vi "FlexMag - 24-03-2023.vi"() -> ()   [LabVIEW 2018] (continued)
                              n10246 = local read "ABORT"() -> (w15652:bool)
                              n10247 = Not(x=w15653) -> (.not. x?=w15651:bool)
                              n10248 = Compound Arithmetic op=OR(w15646, w15652, w15651) -> (w15650:bool)
                            }
                          }
                          frame #2 {
                            n10249 = flat-sequence {
                              frame #0 {
                                n10250 = local write "Cassette_Servo_Speed AO"(0.0 ("Cassette_Servo_Speed AO")) -> ()
                                n10251 = Wait (ms)(milliseconds to wait=u32 100) -> ()  [unwired: 1 out]
                              }
                              frame #1 {
                                n10252 = local write "Cassette_Servo_Speed Set"(TRUE ("Cassette_Servo_Speed Set")) -> ()
                              }
                            }
                          }
                        }
                      }
                      frame True {
                      }
                    }
                  }
                }
              }
              frame #37 {
                n10253 = local read "ch3-4 transfer"() -> (w15663:bool)
                n10254 = case shown="True" w15663 {
                  frame False {
                  }
                  frame True {
                    n10255 = local read "ABORT"() -> (w15664:bool)
                    n10256 = case shown="False" w15664 {
                      frame False {
                        n10257 = local write "trns 3-4 led 17"(TRUE ("trns 1-2 led 1")) -> ()
                        n10258 = Wait (ms)(milliseconds to wait=u32 100) -> ()  [unwired: 1 out]
                      }
                      frame True {
                      }
                    }
                  }
                }
              }
              frame #38 {
                n10259 = local read "ch3-4 transfer"() -> (w15667:bool)
                n10260 = case shown="True" w15667 {
                  frame False {
                  }
                  frame True {
                    n10261 = local read "ABORT"() -> (w15668:bool)
                    n10262 = case shown="False" w15668 {
                      frame False {
                        n10263 = local read "target chamber"() -> (w15669:dbl)
                        n10264 = Equal?(x=w15669, y=4.0) -> (x = y?=w15670:bool)
                        n10265 = case shown="True" w15670 {
                          frame False {
                          }
                          frame True {
                            n10266 = while {
                              i -> [w15676]
                              stop <- w15677 stop-if-true
                              n10267 = Greater Or Equal?(x=w15676, y=100) -> (x >= y?=w15674:bool)
                              n10268 = case shown="True" w15674 {
                                frame False {
                                }
                                frame True {
                                n10269 = local write "Warning Message"("Transfer process canceled!\nCH4 Cassette Fix couldn't reached  to down position" ("Warning Message")) -> ()
                                n10270 = local write "trns error"(TRUE ("TRNS error")) -> ()
                                }
                              }
                              n10271 = local read "CH4_Cst_Fix_Down_DI"() -> (w15672:bool)
                              n10272 = case shown="False" w15672 {
                                tunnel: [FALSE ("CH1_Trns_BP_Left_DO") TRUE ("CH1_Trns_BP_Left_DO")] -> w15673
                                frame False {
                                n10273 = Wait Until Next ms Multiple(millisecond multiple=u32 200) -> ()  [unwired: 1 out]
                                n10274 = local write "CH4_Cst_Fix_DO"(TRUE ("TRNS error")) -> ()
                                }
                                frame True {
                                }
                              }
                              n10275 = local read "ch3-4 transfer"() -> (w15680:bool)
                              n10276 = local read "ABORT"() -> (w15679:bool)
                              n10277 = Not(x=w15680) -> (.not. x?=w15678:bool)
                              n10278 = Compound Arithmetic op=OR(w15673, w15679, w15678) -> (w15677:bool)
                            }
                          }
                        }
                      }
                      frame True {
                      }
                    }
                  }
                }
              }
              frame #39 {
                n10279 = local read "ch3-4 transfer"() -> (w15687:bool)
                n10280 = case shown="True" w15687 {
                  frame False {
                  }
                  frame True {
                    n10281 = local read "ABORT"() -> (w15688:bool)
                    n10282 = case shown="False" w15688 {
                      frame False {
                        n10283 = local write "trns 3-4 led 18"(TRUE ("trns 1-2 led 1")) -> ()
                        n10284 = Wait (ms)(milliseconds to wait=u32 100) -> ()  [unwired: 1 out]
                      }
                      frame True {
                      }
                    }
                  }
                }
              }
              frame #40 {
                n10285 = local read "ch3-4 transfer"() -> (w15691:bool)
                n10286 = case shown="True" w15691 {
                  frame False {
                  }
                  frame True {
                    n10287 = local read "ABORT"() -> (w15692:bool)
                    n10288 = case shown="False" w15692 {
                      frame False {
                        n10289 = while {
                          i -> [w15697]
                          stop <- w15698 stop-if-true
                          n10290 = Greater Or Equal?(x=w15697, y=100) -> (x >= y?=w15695:bool)
                          n10291 = case shown="True" w15695 {
                            frame False {
                            }
                            frame True {
                              n10292 = local write "Warning Message"("Transfer process canceled!\nCH3 Trns Bp Left coulnt't be closed" ("Warning Message")) -> ()
                              n10293 = local write "trns error"(TRUE ("TRNS error")) -> ()
                            }
                          }
                          n10294 = local read "CH3_Trns_BP_Left_DI"() -> (w15693:bool)
                          n10295 = case shown="True" w15693 {
                            tunnel: [TRUE ("CH1_Trns_BP_Left_DO") FALSE ("CH1_Trns_BP_Left_DO")] -> w15694
                            frame False {
                            }
                            frame True {
                              n10296 = Wait Until Next ms Multiple(millisecond multiple=u32 200) -> ()  [unwired: 1 out]
                              n10297 = local write "CH3_Trns_BP_Left_DO"(FALSE ("TRNS error")) -> ()
                            }
                          }
                          n10298 = local read "ch3-4 transfer"() -> (w15701:bool)
                          n10299 = local read "ABORT"() -> (w15700:bool)
                          n10300 = Not(x=w15701) -> (.not. x?=w15699:bool)
                          n10301 = Compound Arithmetic op=OR(w15694, w15700, w15699) -> (w15698:bool)
                        }
                      }
                      frame True {
                      }
                    }
                  }
                }
              }
              frame #41 {
                n10302 = local read "ch3-4 transfer"() -> (w15708:bool)
                n10303 = case shown="True" w15708 {
                  frame False {
                  }
                  frame True {
                    n10304 = local read "ABORT"() -> (w15709:bool)
                    n10305 = case shown="False" w15709 {
                      frame False {
                        n10306 = local write "trns 3-4 led 19"(TRUE ("trns 1-2 led 1")) -> ()
                        n10307 = Wait (ms)(milliseconds to wait=u32 100) -> ()  [unwired: 1 out]
                      }
                      frame True {
                      }
                    }
                  }
                }
              }
              frame #42 {
                n10308 = local read "ch3-4 transfer"() -> (w15712:bool)
                n10309 = case shown="True" w15712 {
                  frame False {
                  }
                  frame True {
                    n10310 = local read "ABORT"() -> (w15713:bool)
                    n10311 = case shown="False" w15713 {
                      frame False {
                        n10312 = while {
                          i -> [w15718]
                          stop <- w15719 stop-if-true
                          n10313 = Greater Or Equal?(x=w15718, y=100) -> (x >= y?=w15716:bool)
                          n10314 = case shown="True" w15716 {
                            frame False {
                            }
                            frame True {
                              n10315 = local write "Warning Message"("Transfer process canceled!\nCH4 Trns Bp Right coulnt't be closed" ("Warning Message")) -> ()
                              n10316 = local write "trns error"(TRUE ("TRNS error")) -> ()
                            }
                          }
                          n10317 = local read "CH4_Trns_BP_Right_DI"() -> (w15714:bool)
                          n10318 = case shown="True" w15714 {
                            tunnel: [TRUE ("CH1_Trns_BP_Left_DO") FALSE ("CH1_Trns_BP_Left_DO")] -> w15715
                            frame False {
                            }
                            frame True {
                              n10319 = local write "CH4_Trns_BP_Right_DO"(FALSE ("TRNS error")) -> ()
                              n10320 = Wait Until Next ms Multiple(millisecond multiple=u32 200) -> ()  [unwired: 1 out]
                            }
                          }
                          n10321 = local read "ch3-4 transfer"() -> (w15722:bool)
                          n10322 = local read "ABORT"() -> (w15721:bool)
                          n10323 = Not(x=w15722) -> (.not. x?=w15720:bool)
                          n10324 = Compound Arithmetic op=OR(w15715, w15721, w15720) -> (w15719:bool)
                        }
                      }
                      frame True {
                      }
                    }
                  }
                }
              }
              frame #43 {
                n10325 = local read "ch3-4 transfer"() -> (w15729:bool)
                n10326 = case shown="True" w15729 {
                  frame False {
                  }
                  frame True {
                    n10327 = local read "ABORT"() -> (w15730:bool)
                    n10328 = case shown="False" w15730 {
                      frame False {
                        n10329 = local write "trns 3-4 led 20"(TRUE ("trns 1-2 led 1")) -> ()
                        n10330 = Wait (ms)(milliseconds to wait=u32 100) -> ()  [unwired: 1 out]
                      }
                      frame True {
                      }
                    }
                  }
                }
              }
              frame #44 {
                n10331 = local read "ch3-4 transfer"() -> (w15733:bool)
                n10332 = case shown="True" w15733 {
                  frame False {
                  }
                  frame True {
                    n10333 = local read "ABORT"() -> (w15734:bool)
                    n10334 = case shown="False" w15734 {
                      frame False {
                        n10335 = stacked-sequence {
                          frame #0 {
                            n10336 = local read "ch3-4 transfer"() -> (w15735:bool)
                            n10337 = case shown="True" w15735 {
                              frame False {
                              }
                              frame True {
                                n10338 = local write "CH3_Trns_GV_Open_DO"(FALSE ("trns clear")) -> ()
                              }
                            }
                          }
                          frame #1 {
                            n10339 = while {
                              i -> [w15741]
                              stop <- w15742 stop-if-true
                              n10340 = Greater Or Equal?(x=w15741, y=600) -> (x >= y?=w15739:bool)
                              n10341 = case shown="True" w15739 {
                                frame False {
                                }
                                frame True {
                                n10342 = local write "Warning Message"("Transfer process canceled!\nCH3-CH4 Trns GV couldn't be closed" ("Warning Message")) -> ()
                                n10343 = local write "trns error"(TRUE ("TRNS error")) -> ()
                                }
                              }
                              n10344 = local read "CH3_Trns_Gv_Close_DI"() -> (w15737:bool)
                              n10345 = case shown="False" w15737 {
                                tunnel: [FALSE ("CH1_Trns_BP_Left_DO") TRUE ("CH1_Trns_BP_Left_DO")] -> w15738
                                frame False {
                                n10346 = local write "CH3_Trns_GV_Close_DO"(TRUE ("TRNS error")) -> ()
                                n10347 = Wait Until Next ms Multiple(millisecond multiple=u32 200) -> ()  [unwired: 1 out]
                                }
                                frame True {
                                }
                              }
                              n10348 = local read "ch3-4 transfer"() -> (w15745:bool)
                              n10349 = local read "ABORT"() -> (w15744:bool)
                              n10350 = Not(x=w15745) -> (.not. x?=w15743:bool)
                              n10351 = Compound Arithmetic op=OR(w15738, w15744, w15743) -> (w15742:bool)
                            }
                          }
                        }
                      }
                      frame True {
                      }
                    }
                  }
                }
              }
              frame #45 {
                n10352 = local read "ch3-4 transfer"() -> (w15752:bool)
                n10353 = case shown="True" w15752 {
                  frame False {
                  }
                  frame True {
                    n10354 = local read "ABORT"() -> (w15753:bool)
                    n10355 = case shown="False" w15753 {
                      frame False {
                        n10356 = local write "trns 3-4 led 21"(TRUE ("trns 1-2 led 1")) -> ()
                        n10357 = Wait (ms)(milliseconds to wait=u32 100) -> ()  [unwired: 1 out]
                      }
                      frame True {
                      }
                    }
                  }
                }
              }
              frame #46 {
                n10358 = local read "ch3-4 transfer"() -> (w15756:bool)
                n10359 = case shown="True" w15756 {
                  frame False {
                  }
                  frame True {
                    n10360 = local read "ABORT"() -> (w15757:bool)
                    n10361 = case shown="False" w15757 {
                      frame False {
                        n10362 = local read "target chamber"() -> (w15758:dbl)
                        n10363 = Equal?(x=w15758, y=4.0) -> (x = y?=w15759:bool)
                        n10364 = case shown="True" w15759 {
                          frame False {
                          }
                          frame True {
                            n10365 = stacked-sequence {
                              frame #0 {
                                n10366 = local read "ch3-4 transfer"() -> (w15761:bool)
                                n10367 = case shown="True" w15761 {
                                frame False {
                                }
                                frame True {
                                n10368 = local write "CH4_PetCool_Up_DO"(FALSE ("trns clear")) -> ()
                                }
                                }
                              }
                              frame #1 {
                                n10369 = while {
                                i -> [w15767]
                                stop <- w15768 stop-if-true
                                n10370 = Greater Or Equal?(x=w15767, y=300) -> (x >= y?=w15765:bool)
                                n10371 = case shown="True" w15765 {
                                frame False {
                                }
                                frame True {
                                n10372 = local write "Warning Message"("Transfer process canceled!\nCH4 Petcool couldn't be down" ("Warning Message")) -> ()
                                n10373 = local write "trns error"(TRUE ("TRNS error")) -> ()
                                }
                                }
                                n10374 = local read "CH4_PetCool_Down_DI"() -> (w15763:bool)
                                n10375 = case shown="False" w15763 {
                                tunnel: [FALSE ("CH1_Trns_BP_Left_DO") TRUE ("CH1_Trns_BP_Left_DO")] -> w15764
                                frame False {
                                n10376 = local write "CH4_PetCool_Down_DO"(TRUE ("TRNS error")) -> ()
                                n10377 = Wait Until Next ms Multiple(millisecond multiple=u32 200) -> ()  [unwired: 1 out]
                                }
                                frame True {
                                }
                                }
                                n10378 = local read "ch3-4 transfer"() -> (w15771:bool)
                                n10379 = local read "ABORT"() -> (w15770:bool)
                                n10380 = Not(x=w15771) -> (.not. x?=w15769:bool)
                                n10381 = Compound Arithmetic op=OR(w15764, w15770, w15769) -> (w15768:bool)
                                }
                              }
                            }
                          }
                        }
                      }
                      frame True {
                      }
                    }
                  }
                }
              }
              frame #47 {
                n10382 = local read "ch3-4 transfer"() -> (w15778:bool)
                n10383 = case shown="True" w15778 {
                  frame False {
                  }
                  frame True {
                    n10384 = local read "ABORT"() -> (w15779:bool)
                    n10385 = case shown="False" w15779 {
                      frame False {
                        n10386 = local write "trns 3-4 led 22"(TRUE ("trns 1-2 led 1")) -> ()
                        n10387 = Wait (ms)(milliseconds to wait=u32 100) -> ()  [unwired: 1 out]
                      }
                      frame True {
                      }
                    }
                  }
                }
              }
              frame #48 {
                n10388 = local read "ch3-4 transfer"() -> (w15782:bool)
                n10389 = case shown="True" w15782 {
                  frame False {
                  }
                  frame True {
                    n10390 = local read "ABORT"() -> (w15783:bool)
                    n10391 = case shown="False" w15783 {
                      frame False {
                        n10392 = local read "target chamber"() -> (w15785:dbl)
                        n10393 = Equal?(x=w15785, y=4.0) -> (x = y?=w15784:bool)
                        n10394 = case shown="True" w15784 {
                          frame False {
                          }
                          frame True {
                            n10395 = stacked-sequence {
                              frame #0 {
                                n10396 = local read "ch3-4 transfer"() -> (w15787:bool)
                                n10397 = case shown="True" w15787 {
                                frame False {
                                }
                                frame True {
                                n10398 = local write "CH4_SRV1_Piston_Back_DO"(FALSE ("trns clear")) -> ()
                                }
                                }
                              }
                              frame #1 {
                                n10399 = while {
                                i -> [w15793]
                                stop <- w15794 stop-if-true
                                n10400 = Greater Or Equal?(x=w15793, y=200) -> (x >= y?=w15791:bool)
                                n10401 = case shown="True" w15791 {
                                frame False {
                                }
                                frame True {
                                n10402 = local write "Warning Message"("Transfer process canceled!\nCH4 Servo Piston couldn't be forward" ("Warning Message")) -> ()
                                n10403 = local write "trns error"(TRUE ("TRNS error")) -> ()
                                }
                                }
                                n10404 = local read "CH4_SRV1_Piston_For_DI"() -> (w15789:bool)
                                n10405 = case shown="False" w15789 {
                                tunnel: [FALSE ("CH1_Trns_BP_Left_DO") TRUE ("CH1_Trns_BP_Left_DO")] -> w15790
                                frame False {
                                n10406 = local write "CH4_SRV1_Piston_For_DO"(TRUE ("TRNS error")) -> ()
                                n10407 = Wait Until Next ms Multiple(millisecond multiple=u32 200) -> ()  [unwired: 1 out]
                                }
                                frame True {
                                }
                                }
                                n10408 = local read "ch3-4 transfer"() -> (w15797:bool)
                                n10409 = local read "ABORT"() -> (w15796:bool)
                                n10410 = Not(x=w15797) -> (.not. x?=w15795:bool)
                                n10411 = Compound Arithmetic op=OR(w15790, w15796, w15795) -> (w15794:bool)
                                }
                              }
                            }
                          }
                        }
                      }
                      frame True {
                      }
                    }
                  }
                }
              }
              frame #49 {
                n10412 = local read "ch3-4 transfer"() -> (w15804:bool)
                n10413 = case shown="True" w15804 {
                  frame False {
                  }
                  frame True {
                    n10414 = local read "ABORT"() -> (w15805:bool)
                    n10415 = case shown="False" w15805 {
                      frame False {
                        n10416 = local write "trns 3-4 led 23"(TRUE ("trns 1-2 led 1")) -> ()
                        n10417 = Wait (ms)(milliseconds to wait=u32 100) -> ()  [unwired: 1 out]
                      }
                      frame True {
                      }
                    }
                  }
                }
              }
              frame #50 {
                n10418 = local read "ch3-4 transfer"() -> (w15808:bool)
                n10419 = case shown="True" w15808 {
                  frame False {
                  }
                  frame True {
                    n10420 = local read "ABORT"() -> (w15809:bool)
                    n10421 = case shown="False" w15809 {
                      frame False {
                        n10422 = disable-structure shown="Enabled" {
                          frame Disabled {
                            n10423 = stacked-sequence {
                              frame #0 {
                                n10424 = while {
                                i -> [w15814]
                                stop <- w15815 stop-if-true
                                n10425 = Greater Or Equal?(x=w15814, y=100) -> (x >= y?=w15812:bool)
                                n10426 = case shown="True" w15812 {
                                frame False {
                                }
                                frame True {
                                n10427 = local write "Warning Message"("Transfer process canceled!\nRight Slow Sensor problem" ("Warning Message")) -> ()
                                n10428 = local write "trns error"(TRUE ("TRNS error")) -> ()
                                }
                                }
                                n10429 = local read "Cnt_Right_Slow DI"() -> (w15810:bool)
                                n10430 = case shown="True" w15810 {
                                tunnel: [TRUE ("CH1_Trns_BP_Left_DO") FALSE ("CH1_Trns_BP_Left_DO")] -> w15811
                                frame False {
                                }
                                frame True {
                                n10431 = Wait Until Next ms Multiple(millisecond multiple=u32 200) -> ()  [unwired: 1 out]
                                n10432 = local write "Cnt_Right_Slow DO"(FALSE ("TRNS error")) -> ()
                                }
                                }
                                n10433 = local read "ch3-4 transfer"() -> (w15818:bool)
                                n10434 = local read "ABORT"() -> (w15817:bool)
                                n10435 = Not(x=w15818) -> (.not. x?=w15816:bool)
                                n10436 = Compound Arithmetic op=OR(w15811, w15817, w15816) -> (w15815:bool)
                                }
                              }
                              frame #1 {
                                n10437 = while {
                                i -> [w15829]
                                stop <- w15830 stop-if-true
                                n10438 = Greater Or Equal?(x=w15829, y=100) -> (x >= y?=w15827:bool)
                                n10439 = case shown="True" w15827 {
                                frame False {
                                }
                                frame True {
                                n10440 = local write "Warning Message"("Transfer process canceled!\nRight Limit Sensor problem" ("Warning Message")) -> ()
                                n10441 = local write "trns error"(TRUE ("TRNS error")) -> ()
                                }
                                }
                                n10442 = local read "Cnt_Right_Limit DI"() -> (w15825:bool)
                                n10443 = case shown="True" w15825 {
                                tunnel: [TRUE ("CH1_Trns_BP_Left_DO") FALSE ("CH1_Trns_BP_Left_DO")] -> w15826
                                frame False {
                                }
                                frame True {
                                n10444 = Wait Until Next ms Multiple(millisecond multiple=u32 200) -> ()  [unwired: 1 out]
                                n10445 = local write "Cnt_Right_Limit DO"(FALSE ("TRNS error")) -> ()
                                }
                                }
                                n10446 = local read "ch3-4 transfer"() -> (w15833:bool)
                                n10447 = local read "ABORT"() -> (w15832:bool)
                                n10448 = Not(x=w15833) -> (.not. x?=w15831:bool)
                                n10449 = Compound Arithmetic op=OR(w15826, w15832, w15831) -> (w15830:bool)
                                }
                              }
                              frame #2 {
                                n10450 = while {
                                i -> [w15844]
                                stop <- w15845 stop-if-true
                                n10451 = Greater Or Equal?(x=w15844, y=100) -> (x >= y?=w15842:bool)
                                n10452 = case shown="True" w15842 {
                                frame False {
                                }
                                frame True {
                                n10453 = local write "Warning Message"("Transfer process canceled!\nLeft Slow Sensor problem" ("Warning Message")) -> ()
                                n10454 = local write "trns error"(TRUE ("TRNS error")) -> ()
                                }
                                }
                                n10455 = local read "Cnt_Left_Slow DI"() -> (w15840:bool)
                                n10456 = case shown="True" w15840 {
                                tunnel: [TRUE ("CH1_Trns_BP_Left_DO") FALSE ("CH1_Trns_BP_Left_DO")] -> w15841
                                frame False {
                                }
                                frame True {
                                n10457 = Wait Until Next ms Multiple(millisecond multiple=u32 200) -> ()  [unwired: 1 out]
                                n10458 = local write "Cnt_Left_Slow DO"(FALSE ("TRNS error")) -> ()
                                }
                                }
                                n10459 = local read "ch3-4 transfer"() -> (w15848:bool)
                                n10460 = local read "ABORT"() -> (w15847:bool)
                                n10461 = Not(x=w15848) -> (.not. x?=w15846:bool)
                                n10462 = Compound Arithmetic op=OR(w15841, w15847, w15846) -> (w15845:bool)
                                }
                              }
                              frame #3 {
                                n10463 = while {
                                i -> [w15859]
                                stop <- w15860 stop-if-true
                                n10464 = Greater Or Equal?(x=w15859, y=100) -> (x >= y?=w15857:bool)
                                n10465 = case shown="True" w15857 {
                                frame False {
                                }
                                frame True {
                                n10466 = local write "Warning Message"("Transfer process canceled!\nLeft Limit Sensor problem" ("Warning Message")) -> ()
                                n10467 = local write "trns error"(TRUE ("TRNS error")) -> ()
                                }
                                }
                                n10468 = local read "Cnt_Left_Limit DI"() -> (w15855:bool)
                                n10469 = case shown="True" w15855 {
                                tunnel: [TRUE ("CH1_Trns_BP_Left_DO") FALSE ("CH1_Trns_BP_Left_DO")] -> w15856
                                frame False {
                                }
                                frame True {
                                n10470 = Wait Until Next ms Multiple(millisecond multiple=u32 200) -> ()  [unwired: 1 out]
                                n10471 = local write "Cnt_Left_Limit DO"(FALSE ("TRNS error")) -> ()
                                }
                                }
                                n10472 = local read "ch3-4 transfer"() -> (w15863:bool)
                                n10473 = local read "ABORT"() -> (w15862:bool)
                                n10474 = Not(x=w15863) -> (.not. x?=w15861:bool)
                                n10475 = Compound Arithmetic op=OR(w15856, w15862, w15861) -> (w15860:bool)
                                }
                              }
                            }
                          }
                          frame Enabled {
                            w15871 = FALSE
                            w15872 = FALSE
                            n10476 = local write "CH1_Right_Limit_DO"(w15872) -> ()
                            n10477 = local write "CH1_Right_Slow_DO"(w15872) -> ()
                            n10478 = local write "CH2_Right_Limit_DO"(w15872) -> ()
                            n10479 = local write "CH2_Right_Slow_DO"(w15872) -> ()
                            n10480 = local write "CH2_Left_Slow_DO"(w15872) -> ()
                            n10481 = local write "CH2_Left_Limit_DO"(w15872) -> ()
                            n10482 = Wait (ms)(milliseconds to wait=u32 2000) -> ()  [unwired: 1 out]
                            n10483 = local write "CH3_Right_Limit_DO"(w15871) -> ()
                            n10484 = local write "CH3_Right_Slow_DO"(w15871) -> ()
                            n10485 = local write "CH3_Left_Slow_DO"(w15871) -> ()
                            n10486 = local write "CH3_Left_Limit_DO"(w15871) -> ()
                            n10487 = local write "CH4_Left_Limit_DO"(w15871) -> ()
                            n10488 = local write "CH4_Left_Slow_DO"(w15871) -> ()
                          }
                        }
                      }
                      frame True {
                      }
                    }
                  }
                }
              }
              frame #51 {
                n10489 = local read "ch3-4 transfer"() -> (w15873:bool)
                n10490 = case shown="True" w15873 {
                  frame False {
                  }
                  frame True {
                    n10491 = local read "ABORT"() -> (w15874:bool)
                    n10492 = case shown="False" w15874 {
                      frame False {
                        n10493 = local write "trns 3-4 led 24"(TRUE ("trns 1-2 led 17")) -> ()
                        n10494 = Wait (ms)(milliseconds to wait=u32 100) -> ()  [unwired: 1 out]
                      }
                      frame True {
                      }
                    }
                  }
                }
              }
              frame #52 {
                n10495 = local read "ch3-4 transfer"() -> (w15877:bool)
                n10496 = case shown="True" w15877 {
                  frame False {
                  }
                  frame True {
                    n10497 = local read "ABORT"() -> (w15878:bool)
                    n10498 = case shown="False" w15878 {
                      frame False {
                        n10499 = local write "Buzzer DO"(TRUE ("trns 1-2 led 17")) -> ()
                        n10500 = Wait (ms)(milliseconds to wait=u32 3000) -> ()  [unwired: 1 out]
                        n10501 = local write "System Status"("CH3 to CH4  Transfer Completed" ("System Status")) -> ()
                      }
                      frame True {
                      }
                    }
                  }
                }
              }
              frame #53 {
                n10502 = local read "ch3-4 transfer"() -> (w15882:bool)
                n10503 = case shown="True" w15882 {
                  frame False {
                  }
                  frame True {
                    n10504 = local read "ABORT"() -> (w15883:bool)
                    n10505 = case shown="False" w15883 {
                      frame False {
                        w15884 = u16 4 items=["CH1"=1, "CH2"=2, "CH3"=3, "CH4"=4] ("cassette position selection")
                        w15885 = FALSE ("trns 1-2 led 17")
                        n10506 = Wait (ms)(milliseconds to wait=u32 1000) -> ()  [unwired: 1 out]
                        n10507 = local write "cassette position selection"(w15884) -> ()
                        n10508 = local write "ch3-4 transfer"(FALSE ("trns 1-2 led 17")) -> ()
                        n10509 = local write "Buzzer DO"(FALSE ("trns 1-2 led 17")) -> ()
                        n10510 = local write "System Status"("SEMI-AUTOMATIC MODE " ("System Status")) -> ()
                        n10511 = Not(x=w15885) -> (.not. x?=w15886:bool)
                        n10512 = local write "present location"(4.0 ("present location")) -> ()
                        n10513 = local write "casette_ch1_gui"(w15885) -> ()
                        n10514 = local write "casette_ch2_gui"(w15885) -> ()
                        n10515 = local write "casette_ch3_gui"(w15885) -> ()
                        n10516 = local write "casette_ch4_gui"(w15886) -> ()
                      }
                      frame True {
                      }
                    }
                  }
                }
              }
              frame #54 {
              }
            }
          }
          frame True {
          }
        }
      }
      frame 4 {
        n10517 = local read "ABORT"() -> (w15892:bool)
        n10518 = case shown="False" w15892 {
          frame False {
            n10519 = stacked-sequence {
              frame #0 {
                n10520 = local read "ch2-1 transfer"() -> (w15893:bool)
                n10521 = case shown="True" w15893 {
                  frame False {
                  }
                  frame True {
                    n10522 = local read "present location"() -> (w15896:dbl)
                    n10523 = Wait (ms)(milliseconds to wait=u32 100) -> ()  [unwired: 1 out]
                    n10524 = Equal?(x=w15896, y=2.0) -> (x = y?=w15897:bool)
                    n10525 = case shown="True" w15897 {
                      frame False {
                        n10526 = local write "trns error"(TRUE ("TRNS error")) -> ()
                        n10527 = local write "Warning Message"("Transfer process canceled!\nCassette is not in CH2" ("Warning Message")) -> ()
                      }
                      frame True {
                        n10528 = local write "System Status"("CH2 to CH1  Transfer in Progress" ("System Status")) -> ()
                      }
                    }
                  }
                }
              }
              frame #1 {
                n10529 = local read "ch2-1 transfer"() -> (w15901:bool)
                n10530 = case shown="True" w15901 {
                  frame False {
                  }
                  frame True {
                    n10531 = stacked-sequence {
                      frame #0 {
                        n10532 = local read "ABORT"() -> (w15902:bool)
                        n10533 = case shown="False" w15902 {
                          frame False {
                            n10534 = local write "trns pre check"(TRUE ("trns pre check")) -> ()
                          }
                          frame True {
                          }
                        }
                      }
                      frame #1 {
                        n10535 = Wait (ms)(milliseconds to wait=u32 1000) -> ()  [unwired: 1 out]
                      }
                      frame #2 {
                        n10536 = while {
                          i -> [w15910]
                          stop <- w15907 stop-if-true
                          # "10 min"
                          n10537 = local read "trns pre check"() -> (w15914:bool)
                          n10538 = local read "ch2-1 transfer"() -> (w15906:bool)
                          n10539 = local read "ABORT"() -> (w15908:bool)
                          n10540 = Greater Or Equal?(x=w15910, y=u32 2000 ("millisecond multiple")) -> (x >= y?=w15909:bool)
                          n10541 = Not(x=w15914) -> (.not. x?=w15913:bool)
                          n10542 = Not(x=w15906) -> (.not. x?=w15905:bool)
                          n10543 = Compound Arithmetic op=OR(w15909, w15913, w15908, w15905) -> (w15907:bool)
                          n10544 = Wait Until Next ms Multiple(millisecond multiple=u32 300) -> ()  [unwired: 1 out]
                        }
                      }
                    }
                  }
                }
              }
              frame #2 {
                n10545 = local read "ch2-1 transfer"() -> (w15915:bool)
                n10546 = case shown="True" w15915 {
                  frame False {
                  }
                  frame True {
                    n10547 = local read "trns V?"() -> (w15916:bool)
                    n10548 = case shown="True" w15916 {
                      frame False {
                        n10549 = stacked-sequence {
                          frame #0 {
                            n10550 = local read "ABORT"() -> (w15917:bool)
                            n10551 = case shown="False" w15917 {
                              frame False {
                                w15919 = FALSE ("CH1_CH_ATM_DO")
                                n10552 = local write "CH1_CH_ATM_DO"(w15919) -> ()
                                n10553 = local write "CH2_CH_ATM_DO"(w15919) -> ()
                                n10554 = Wait (ms)(milliseconds to wait=u32 3000) -> ()  [unwired: 1 out]
                              }
                              frame True {
                              }
                            }
                          }
                          frame #1 {
                            n10555 = while {
                              i -> [w15922]
                              stop <- w15923 stop-if-true
                              n10556 = Greater Or Equal?(x=w15922, y=200) -> (x >= y?=w15920:bool)
                              n10557 = case shown="True" w15920 {
                                frame False {
                                }
                                frame True {
                                n10558 = local write "Warning Message"("Transfer process canceled!\nChambers should be on Atmosphere Pressure" ("Warning Message")) -> ()
                                n10559 = local write "trns error"(TRUE ("TRNS error")) -> ()
                                }
                              }
                              n10560 = local read "CH1_CH_ATM_DI"() -> (w15927:bool)
                              n10561 = local read "CH2_CH_ATM_DI"() -> (w15926:bool)
                              n10562 = local read "ch2-1 transfer"() -> (w15929:bool)
                              n10563 = local read "ABORT"() -> (w15930:bool)
                              n10564 = Not(x=w15929) -> (.not. x?=w15928:bool)
                              n10565 = And(x=w15927, y=w15926) -> (x .and. y?=w15925:bool)
                              n10566 = Compound Arithmetic op=OR(w15925, w15930, w15928) -> (w15923:bool)
                              n10567 = Wait Until Next ms Multiple(millisecond multiple=u32 300) -> ()  [unwired: 1 out]
                            }
                          }
                        }
                      }
                      frame True {
                        n10568 = local read "ch1 ch pg torr"() -> (w15939:dbl)
                        n10569 = local read "ch2 ch pg torr"() -> (w15936:dbl)
                        n10570 = Greater Or Equal?(x=w15939, y=0.5) -> (x >= y?=w15935:bool)
                        n10571 = Greater Or Equal?(x=w15936, y=0.5) -> (x >= y?=w15934:bool)
                        n10572 = Or(x=w15935, y=w15934) -> (x .or. y?=w15933:bool)
                        n10573 = local write "trns error"(w15933) -> ()
                      }
                    }
                  }
                }
              }
              frame #3 {
                n10574 = local read "ch2-1 transfer"() -> (w15940:bool)
                n10575 = case shown="True" w15940 {
                  frame False {
                  }
                  frame True {
                    n10576 = local read "ABORT"() -> (w15941:bool)
                    n10577 = case shown="False" w15941 {
                      frame False {
                        n10578 = while {
                          i -> [w15946]
                          stop <- w15947 stop-if-true
                          n10579 = Greater Or Equal?(x=w15946, y=100) -> (x >= y?=w15944:bool)
                          n10580 = case shown="True" w15944 {
                            frame False {
                            }
                            frame True {
                              n10581 = local write "trns error"(TRUE ("TRNS error")) -> ()
                              n10582 = local write "Warning Message"("Transfer process canceled!\nCH1 Trns BP Left couln't be opened" ("Warning Message")) -> ()
                            }
                          }
                          n10583 = local read "CH1_Trns_BP_Left_DI"() -> (w15943:bool)
                          n10584 = case shown="False" w15943 {
                            tunnel: [FALSE ("CH1_Trns_BP_Left_DO") TRUE ("CH1_Trns_BP_Left_DO")] -> w15942
                            frame False {
                              n10585 = Wait Until Next ms Multiple(millisecond multiple=u32 200) -> ()  [unwired: 1 out]
                              n10586 = local write "CH1_Trns_BP_Left_DO"(TRUE ("CH1_Trns_BP_Left_DO")) -> ()
                            }
                            frame True {
                            }
                          }
                          n10587 = local read "ch2-1 transfer"() -> (w15950:bool)
                          n10588 = local read "ABORT"() -> (w15949:bool)
                          n10589 = Not(x=w15950) -> (.not. x?=w15948:bool)
                          n10590 = Compound Arithmetic op=OR(w15942, w15949, w15948) -> (w15947:bool)
                        }
                      }
                      frame True {
                      }
                    }
                  }
                }
              }
              frame #4 {
                n10591 = local read "ch2-1 transfer"() -> (w15957:bool)
                n10592 = case shown="True" w15957 {
                  frame False {
                  }
                  frame True {
                    n10593 = local read "ABORT"() -> (w15958:bool)
                    n10594 = case shown="False" w15958 {
                      frame False {
                        n10595 = local write "trns 2-1 led 1"(TRUE ("trns 1-2 led 1")) -> ()
                        n10596 = Wait (ms)(milliseconds to wait=u32 100) -> ()  [unwired: 1 out]
                      }
                      frame True {
                      }
                    }
                  }
                }
              }
              frame #5 {
                n10597 = local read "ch2-1 transfer"() -> (w15961:bool)
                n10598 = case shown="True" w15961 {
                  frame False {
                  }
                  frame True {
                    n10599 = local read "ABORT"() -> (w15962:bool)
                    n10600 = case shown="False" w15962 {
                      frame False {
                        n10601 = while {
                          i -> [w15967]
                          stop <- w15968 stop-if-true
                          n10602 = Greater Or Equal?(x=w15967, y=100) -> (x >= y?=w15965:bool)
                          n10603 = case shown="True" w15965 {
                            frame False {
                            }
                            frame True {
                              n10604 = local write "trns error"(TRUE ("TRNS error")) -> ()
                              n10605 = local write "Warning Message"("Transfer process canceled!\nCH2 Trns BP Right couln't be opened" ("Warning Message")) -> ()
                            }
                          }
                          n10606 = local read "CH2_Trns_BP_Right_DI"() -> (w15964:bool)
                          n10607 = case shown="False" w15964 {
                            tunnel: [FALSE ("CH1_Trns_BP_Left_DO") TRUE ("CH1_Trns_BP_Left_DO")] -> w15963
                            frame False {
                              n10608 = Wait Until Next ms Multiple(millisecond multiple=u32 200) -> ()  [unwired: 1 out]
                              n10609 = local write "CH2_Trns_BP_Right_DO"(TRUE ("CH1_Trns_BP_Left_DO")) -> ()
                            }
                            frame True {
                            }
                          }
                          n10610 = local read "ch2-1 transfer"() -> (w15971:bool)
                          n10611 = local read "ABORT"() -> (w15970:bool)
                          n10612 = Not(x=w15971) -> (.not. x?=w15969:bool)
                          n10613 = Compound Arithmetic op=OR(w15963, w15970, w15969) -> (w15968:bool)
                        }
                      }
                      frame True {
                      }
                    }
                  }
                }
              }
              frame #6 {
                n10614 = local read "ch2-1 transfer"() -> (w15978:bool)
                n10615 = case shown="True" w15978 {
                  frame False {
                  }
                  frame True {
                    n10616 = local read "ABORT"() -> (w15979:bool)
                    n10617 = case shown="False" w15979 {
                      frame False {
                        n10618 = local write "trns 2-1 led 2"(TRUE ("trns 1-2 led 1")) -> ()
                        n10619 = Wait (ms)(milliseconds to wait=u32 100) -> ()  [unwired: 1 out]
                      }
                      frame True {
                      }
                    }
                  }
                }
              }
              frame #7 {
                n10620 = local read "ch2-1 transfer"() -> (w15982:bool)
                n10621 = case shown="True" w15982 {
                  frame False {
                  }
                  frame True {
                    n10622 = local read "ABORT"() -> (w15983:bool)
                    n10623 = case shown="False" w15983 {
                      frame False {
                        n10624 = stacked-sequence {
                          frame #0 {
                            n10625 = local write "CH1_Trns_Gv_Close_DO"(FALSE ("CH1_Trns_Gv_Close_DO")) -> ()
                            n10626 = Wait (ms)(milliseconds to wait=u32 100) -> ()  [unwired: 1 out]
                          }
                          frame #1 {
                            n10627 = while {
                              i -> [w15990]
                              stop <- w15991 stop-if-true
                              n10628 = Greater Or Equal?(x=w15990, y=600) -> (x >= y?=w15988:bool)
                              n10629 = case shown="True" w15988 {
                                frame False {
                                }
                                frame True {
                                n10630 = local write "trns error"(TRUE ("TRNS error")) -> ()
                                n10631 = local write "Warning Message"("Transfer process canceled!\nCH1-CH2 Trns GV couldn't be opened" ("Warning Message")) -> ()
                                }
                              }
                              n10632 = local read "CH1_Trns_Gv_Open_DI"() -> (w15987:bool)
                              n10633 = case shown="False" w15987 {
                                tunnel: [FALSE ("CH1_Trns_BP_Left_DO") TRUE ("CH1_Trns_BP_Left_DO")] -> w15986
                                frame False {
                                n10634 = local write "CH1_Trns_Gv_Open_DO"(TRUE ("CH1_Trns_BP_Left_DO")) -> ()
                                n10635 = Wait Until Next ms Multiple(millisecond multiple=u32 200) -> ()  [unwired: 1 out]
                                }
                                frame True {
                                }
                              }
                              n10636 = local read "ch2-1 transfer"() -> (w15994:bool)
                              n10637 = local read "ABORT"() -> (w15993:bool)
                              n10638 = Not(x=w15994) -> (.not. x?=w15992:bool)
                              n10639 = Compound Arithmetic op=OR(w15986, w15993, w15992) -> (w15991:bool)
                            }
                          }
                        }
                      }
                      frame True {
                      }
                    }
                  }
                }
              }
              frame #8 {
                n10640 = local read "ch2-1 transfer"() -> (w16001:bool)
                n10641 = case shown="True" w16001 {
                  frame False {
                  }
                  frame True {
                    n10642 = local read "ABORT"() -> (w16002:bool)
                    n10643 = case shown="False" w16002 {
                      frame False {
                        n10644 = local write "trns 2-1 led 3"(TRUE ("trns 1-2 led 1")) -> ()
                        n10645 = Wait (ms)(milliseconds to wait=u32 100) -> ()  [unwired: 1 out]
                      }
                      frame True {
                      }
                    }
                  }
                }
              }
              frame #9 {
                n10646 = local read "ch2-1 transfer"() -> (w16005:bool)
                n10647 = case shown="True" w16005 {
                  frame False {
                  }
                  frame True {
                    n10648 = local read "ABORT"() -> (w16006:bool)
                    n10649 = case shown="False" w16006 {
                      frame False {
                        n10650 = while {
                          i -> [w16011]
                          stop <- w16012 stop-if-true
                          n10651 = Greater Or Equal?(x=w16011, y=100) -> (x >= y?=w16009:bool)
                          n10652 = case shown="True" w16009 {
                            frame False {
                            }
                            frame True {
                              n10653 = local write "trns error"(TRUE ("TRNS error")) -> ()
                              n10654 = local write "Warning Message"("Transfer process canceled!\nCH1 TGV Control Problem" ("Warning Message")) -> ()
                            }
                          }
                          n10655 = local read "CH1_TGV_Control_DI"() -> (w16008:bool)
                          n10656 = case shown="True" w16008 {
                            tunnel: [TRUE ("CH1_Trns_BP_Left_DO") FALSE ("CH1_Trns_BP_Left_DO")] -> w16007
                            frame False {
                            }
                            frame True {
                              n10657 = Wait Until Next ms Multiple(millisecond multiple=u32 200) -> ()  [unwired: 1 out]
                              n10658 = local write "CH1_TGV_Control_DO"(FALSE ("CH1_Trns_BP_Left_DO")) -> ()
                            }
                          }
                          n10659 = local read "ch2-1 transfer"() -> (w16015:bool)
                          n10660 = local read "ABORT"() -> (w16014:bool)
                          n10661 = Not(x=w16015) -> (.not. x?=w16013:bool)
                          n10662 = Compound Arithmetic op=OR(w16007, w16014, w16013) -> (w16012:bool)
                        }
                      }
                      frame True {
                      }
                    }
                  }
                }
              }
              frame #10 {
                n10663 = local read "ch2-1 transfer"() -> (w16022:bool)
                n10664 = case shown="True" w16022 {
                  frame False {
                  }
                  frame True {
                    n10665 = local read "ABORT"() -> (w16023:bool)
                    n10666 = case shown="False" w16023 {
                      frame False {
                        n10667 = local write "trns 2-1 led 4"(TRUE ("trns 1-2 led 1")) -> ()
                        n10668 = Wait (ms)(milliseconds to wait=u32 100) -> ()  [unwired: 1 out]
                      }
                      frame True {
                      }
                    }
                  }
                }
              }
              frame #11 {
                n10669 = local read "ch2-1 transfer"() -> (w16026:bool)
                n10670 = case shown="True" w16026 {
                  frame False {
                  }
                  frame True {
                    n10671 = local read "ABORT"() -> (w16027:bool)
                    n10672 = case shown="False" w16027 {
                      frame False {
                        n10673 = while {
                          i -> [w16032]
                          stop <- w16033 stop-if-true
                          n10674 = local read "CH2_Trns_Interlock_DI"() -> (w16028:bool)
                          n10675 = Greater Or Equal?(x=w16032, y=100) -> (x >= y?=w16030:bool)
                          n10676 = case shown="True" w16030 {
                            frame False {
                            }
                            frame True {
                              n10677 = local write "Warning Message"("Transfer process canceled!\nCH2 Interlock problem" ("Warning Message")) -> ()
                              n10678 = local write "trns error"(TRUE ("TRNS error")) -> ()
                            }
                          }
                          n10679 = case shown="False" w16028 {